vi "SO2 Span Gas Preparation.vi"() -> ()   [LabVIEW 2014]
panel:
  out "CO preflight Des 1":string="SO2 Ground Span Gas Preflight Checks - DO NOT GET DISTRACTED!\n\n1. Check quick connect male body is connected to 'chem 1' gas line.\n\n2. Open cylinder valve 1.\n\n3. Set regulator (V2) to deliver at 3 bar.\n\n4. Open regulator valve 3 (anti-clockwise).\n\n5. Close cylinder valve 1.\n"
  in  "Exit":bool
  # "V3"
  # "V2"
  # "V1"
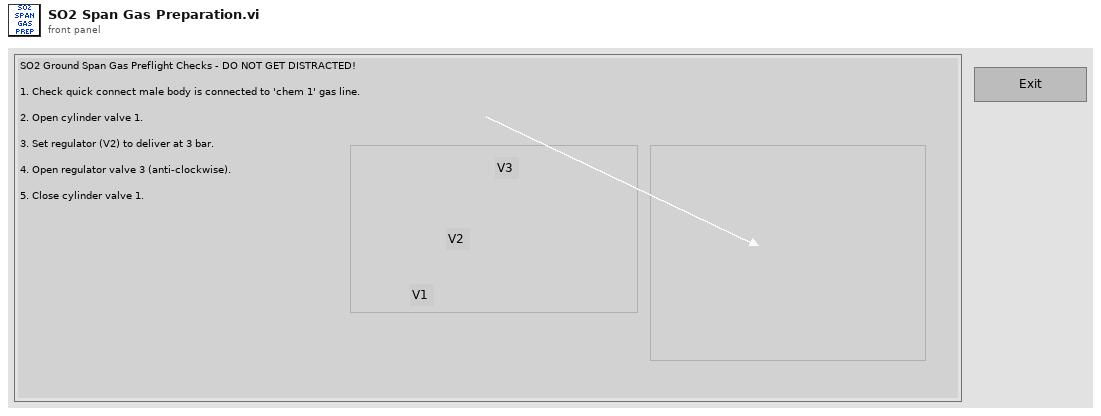
[diagram p1: front panel]
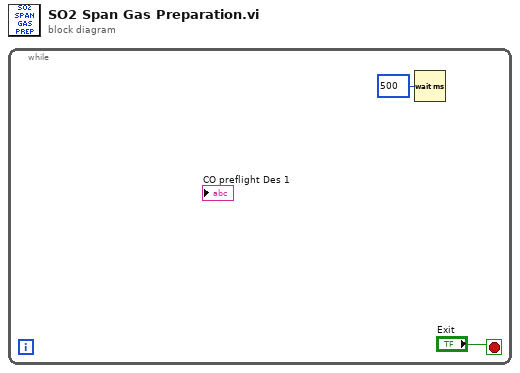
[diagram p0: block diagram]
diagram:
  n1 = while {
    stop <- "Exit" stop-if-true
    n2 = Wait (ms)(milliseconds to wait=u32 500) -> ()  [unwired: 1 out]
  }
